vi "phasemap_slope.vi"() -> ()   [LabVIEW 2011]
uses:
  global_vars.vi
  <userlib>/_OpenG.lib/file/file.llb/Build Path - Traditional__ogtk.vi
panel:
  out "select_col 2":dbl[](array[numeric])
  out "check1":dbl[][](array[numeric])
  out "select_col":dbl[](array[numeric])
  in  "pick col":i32(slide)=225 min=0 scale=0.0..999.0
  out "Y_Displacement (px)":i32[](graph)
  out "X_Displacement (px)":i32[](graph)
  out "x_px_dist":i32[](array[numeric])
  out "Min_values":dbl[](array[numeric])
  out "Min_indices":dbl[](array[numeric])
  out "M_test":dbl[][](array[numeric])
  out "u8_ar_phase map 2":u8[][](array[numeric])
  out "nd_ar_unwrapped_px_ar":dbl[][](array[numeric])
  out "df_ar_unwrapped_px_ar":dbl[][](array[numeric])
  out "Ndist_img":u8[][][](array[numeric])
  in  "read files no-dist":bool
  in  "normalize":bool=TRUE
  out "Phase Line (unwrapped)":dbl[](graph)=[0.0, 0.6594827586206897, 1.0991379310344829, 1.3189655172413794, 1.978448275862069, 2.418103448275862, 2.8577586206896552, 3.2974137931034484, 3.7370689655172415, 4.176724137931035, 4.616379310344827, 5.056034482758621, 5.495689655172414, 5.935344827586207, 6.375, 6.814655172413794, 7.254310344827586, 7.69396551724138, 8.133620689655173, 8.573275862068966, 9.01293103448276, 9.452586206896552, 9.892241379310345, 10.331896551724139, 10.551724137931036, 10.991379310344827, 11.431034482758621, 11.870689655172415, 12.310344827586208, 12.75, 13.189655172413794, 13.629310344827587, 14.068965517241379, 14.508620689655173, 14.948275862068966, 15.38793103448276, 15.607758620689657, 16.04741379310345, 16.487068965517242, 16.926724137931036, 17.36637931034483, 17.806034482758623, 18.02586206896552, 18.46551724137931, 18.905172413793103, 19.344827586206897, 19.78448275862069, 20.224137931034484, 20.44396551724138, 21.10344827586207, 21.323275862068968, 21.762931034482758, 22.20258620689655, 22.642241379310345, 22.862068965517242, 23.301724137931036, 23.74137931034483, 24.181034482758623, 24.620689655172416, 24.84051724137931, 25.280172413793103, 25.719827586206897, 26.15948275862069, 26.379310344827587, 26.81896551724138, 27.258620689655174, 27.47844827586207, 27.918103448275865, 28.357758620689655, 28.57758620689655, 29.017241379310345, 29.45689655172414, 29.896551724137932, 30.11637931034483, 30.556034482758623, 30.995689655172416, 31.435344827586206, 31.655172413793103, 32.0948275862069, 32.314655172413794, 32.75431034482759, 33.19396551724138, 33.41379310344828, 33.85344827586207, 34.293103448275865, 34.51293103448276, 34.952586206896555, 35.39224137931035, 35.612068965517246, 36.05172413793104, 36.491379310344826, 36.71120689655172, 37.150862068965516, 37.37068965517241, 37.810344827586206, 38.25, 38.4698275862069, 38.90948275862069, 39.12931034482759, 39.56896551724138, 40.008620689655174, 40.22844827586207, 40.668103448275865, 40.88793103448276, 41.327586206896555, 41.54741379310345, 41.987068965517246, 42.42672413793104, 42.646551724137936, 42.86637931034483, 43.30603448275862, 43.74568965517241, 43.96551724137931, 44.4051724137931, 44.625, 45.064655172413794, 45.28448275862069, 45.724137931034484, 45.94396551724138, 46.383620689655174, 46.60344827586207, 47.043103448275865, 47.26293103448276, 47.702586206896555, 47.92241379310345, 48.362068965517246, 48.58189655172414, 49.021551724137936, 49.24137931034483, 49.46120689655173, 49.900862068965516, 50.12068965517241, 50.560344827586206, 50.7801724137931, 51.2198275862069, 51.439655172413794, 51.87931034482759, 52.099137931034484, 52.53879310344828, 52.758620689655174, 52.97844827586207, 53.418103448275865, 53.63793103448276, 54.077586206896555, 54.29741379310345, 54.51724137931035, 54.95689655172414, 55.17672413793104, 55.396551724137936, 55.83620689655173, 56.056034482758626, 56.49568965517241, 56.71551724137931, 57.1551724137931, 57.375, 57.5948275862069, 57.814655172413794, 58.25431034482759, 58.474137931034484, 58.69396551724138, 59.133620689655174, 59.35344827586207, 59.793103448275865, 60.01293103448276, 60.23275862068966, 60.67241379310345, 60.89224137931035, 61.112068965517246, 61.33189655172414, 61.771551724137936, 61.99137931034483, 62.431034482758626, 62.65086206896552, 62.87068965517241, 63.09051724137931, 63.310344827586206, 63.75, 63.9698275862069, 64.1896551724138, 64.62931034482759, 64.84913793103449, 65.06896551724138, 65.28879310344828, 65.72844827586208, 65.94827586206897, 66.16810344827586, 66.60775862068965, 66.82758620689656, 67.04741379310344, 67.26724137931035, 67.48706896551724, 67.92672413793103, 68.14655172413794, 68.36637931034483, 68.58620689655173, 68.80603448275862, 69.24568965517241, 69.46551724137932, 69.6853448275862, 69.90517241379311, 70.125, 70.5646551724138, 70.7844827586207, 71.00431034482759, 71.22413793103449, 71.66379310344828, 71.88362068965517, 72.10344827586208, 72.32327586206897, 72.54310344827587, 72.76293103448276, 73.20258620689656, 73.42241379310344, 73.64224137931035, 73.86206896551724, 74.08189655172414, 74.30172413793103, 74.74137931034483, 74.96120689655173, 75.18103448275862, 75.40086206896552, 75.62068965517241, 75.84051724137932, 76.0603448275862, 76.5, 76.7198275862069, 76.9396551724138, 77.1594827586207, 77.37931034482759, 77.59913793103449, 77.81896551724138, 78.03879310344828, 78.25862068965517, 78.47844827586208, 78.91810344827587, 79.13793103448276, 79.13793103448276, 79.57758620689656, 79.79741379310344, 80.01724137931035, 80.23706896551724, 80.45689655172414, 80.67672413793103, 80.89655172413794, 81.11637931034483, 81.33620689655173, 81.55603448275862, 81.77586206896552, 82.21551724137932, 82.4353448275862, 82.65517241379311, 82.875, 83.0948275862069, 83.3146551724138, 83.5344827586207, 83.75431034482759, 83.97413793103449, 84.19396551724138, 84.41379310344828, 84.63362068965517, 84.85344827586208, 85.07327586206897, 85.29310344827587, 85.51293103448276, 85.73275862068967, 85.73275862068967, 85.95258620689656, 86.17241379310344, 86.39224137931035, 86.61206896551724, 86.83189655172414, 87.05172413793103, 87.27155172413794, 87.49137931034483, 87.71120689655173, 87.93103448275862, 88.15086206896552, 88.37068965517241, 88.59051724137932, 88.8103448275862, 89.03017241379311, 89.25, 89.4698275862069, 89.6896551724138, 89.9094827586207, 90.12931034482759, 90.34913793103449, 90.56896551724138, 90.78879310344828, 91.00862068965517, 91.22844827586208, 91.44827586206897, 91.44827586206897, 91.88793103448276, 91.88793103448276, 92.32758620689656, 92.54741379310344, 92.54741379310344, 92.76724137931035, 92.98706896551724, 93.20689655172414, 93.42672413793103, 93.64655172413794, 93.86637931034483, 94.08620689655173, 94.30603448275862, 94.52586206896552, 94.52586206896552, 94.96551724137932, 94.96551724137932, 95.1853448275862, 95.40517241379311, 95.625, 95.8448275862069, 96.0646551724138, 96.2844827586207, 96.50431034482759, 96.72413793103449, 96.72413793103449, 96.94396551724138, 97.16379310344828, 97.38362068965517, 97.60344827586208, 97.82327586206897, 98.04310344827587, 98.26293103448276, 98.48275862068967, 98.48275862068967, 98.70258620689656, 98.92241379310346, 99.14224137931035, 99.36206896551724, 99.58189655172414, 99.80172413793103, 100.02155172413794, 100.02155172413794, 100.24137931034483, 100.46120689655173, 100.68103448275862, 100.90086206896552, 101.12068965517241, 101.34051724137932, 101.34051724137932, 101.5603448275862, 101.78017241379311, 102.0, 102.2198275862069, 102.4396551724138, 102.4396551724138, 102.6594827586207, 102.87931034482759, 103.09913793103449, 103.31896551724138, 103.53879310344828, 103.53879310344828, 103.75862068965517, 103.97844827586208, 104.19827586206897, 104.41810344827587, 104.63793103448276, 104.63793103448276, 104.85775862068967, 105.07758620689656, 105.29741379310346, 105.29741379310346, 105.51724137931035, 105.73706896551724, 105.95689655172414, 106.17672413793103, 106.39655172413794, 106.61637931034483, 106.61637931034483, 106.83620689655173, 107.05603448275862, 107.05603448275862, 107.27586206896552, 107.49568965517241, 107.71551724137932, 107.9353448275862, 108.15517241379311, 108.375, 108.375, 108.5948275862069, 108.8146551724138, 109.0344827586207, 109.0344827586207, 109.25431034482759, 109.47413793103449, 109.69396551724138, 109.91379310344828, 109.91379310344828, 110.13362068965517, 110.35344827586208, 110.57327586206897, 110.57327586206897, 110.79310344827587, 111.01293103448276, 111.23275862068967, 111.23275862068967, 111.45258620689656, 111.67241379310346, 111.89224137931035, 112.11206896551725, 112.11206896551725, 112.33189655172414, 112.55172413793103, 112.77155172413794, 112.99137931034483, 112.99137931034483, 113.21120689655173, 113.43103448275862, 113.43103448275862, 113.65086206896552, 113.87068965517241, 114.09051724137932, 114.3103448275862, 114.3103448275862, 114.53017241379311, 114.75, 114.75, 114.9698275862069, 115.1896551724138, 115.4094827586207, 115.4094827586207, 115.62931034482759, 115.84913793103449, 116.06896551724138, 116.28879310344828, 116.28879310344828, 116.50862068965517, 116.72844827586208, 116.72844827586208, 116.94827586206897, 117.16810344827587, 117.38793103448276, 117.38793103448276, 117.60775862068967, 117.82758620689656, 117.82758620689656, 118.26724137931035, 118.26724137931035, 118.48706896551725, 118.70689655172414, 118.70689655172414, 118.92672413793103, 118.92672413793103, 119.14655172413794, 119.36637931034483, 119.58620689655173, 119.80603448275862, 119.80603448275862, 120.02586206896552, 120.24568965517241, 120.46551724137932, 120.46551724137932, 120.6853448275862, 120.90517241379311, 120.90517241379311, 121.125, 121.3448275862069, 121.5646551724138, 121.5646551724138, 121.7844827586207, 122.00431034482759, 122.22413793103449, 122.22413793103449, 122.44396551724138, 122.66379310344828, 122.66379310344828, 122.88362068965517, 123.10344827586208, 123.32327586206897, 123.32327586206897, 123.54310344827587, 123.76293103448276, 123.76293103448276, 123.98275862068967, 124.20258620689656, 124.20258620689656, 124.42241379310346, 124.64224137931035, 124.86206896551725, 124.86206896551725, 125.08189655172414, 125.30172413793105, 125.30172413793105, 125.52155172413794, 125.74137931034483, 125.96120689655173, 125.96120689655173, 126.18103448275862, 126.40086206896552, 126.62068965517241, 126.62068965517241, 126.84051724137932, 127.0603448275862, 127.28017241379311, 127.28017241379311, 127.5, 127.5, 127.7198275862069, 127.9396551724138, 128.1594827586207, 128.1594827586207, 128.3793103448276, 128.59913793103448, 128.8189655172414, 128.8189655172414, 129.03879310344828, 129.25862068965517, 129.25862068965517, 129.47844827586206, 129.69827586206898, 129.91810344827587, 129.91810344827587, 130.13793103448276, 130.35775862068965, 130.57758620689657, 130.57758620689657, 130.79741379310346, 130.79741379310346, 131.01724137931035, 131.23706896551724, 131.45689655172416, 131.45689655172416, 131.67672413793105, 131.89655172413794, 132.11637931034483, 132.11637931034483, 132.33620689655172, 132.55603448275863, 132.55603448275863, 132.77586206896552, 132.9956896551724, 133.2155172413793, 133.2155172413793, 133.43534482758622, 133.6551724137931, 133.6551724137931, 133.875, 134.0948275862069, 134.3146551724138, 134.3146551724138, 134.5344827586207, 134.7543103448276, 134.7543103448276, 134.97413793103448, 135.1939655172414, 135.41379310344828, 135.41379310344828, 135.63362068965517, 135.85344827586206, 136.07327586206898, 136.07327586206898, 136.29310344827587, 136.51293103448276, 136.51293103448276, 136.73275862068965, 136.95258620689657, 137.17241379310346, 137.17241379310346, 137.39224137931035, 137.61206896551724, 137.83189655172416, 138.05172413793105, 138.05172413793105, 138.27155172413794, 138.49137931034483, 138.71120689655172, 138.71120689655172, 138.93103448275863, 139.15086206896552, 139.15086206896552, 139.3706896551724, 139.5905172413793, 139.81034482758622, 139.81034482758622, 140.0301724137931, 140.25, 140.25, 140.4698275862069, 140.6896551724138, 140.9094827586207, 141.1293103448276, 141.1293103448276, 141.34913793103448, 141.5689655172414, 141.78879310344828, 141.78879310344828, 142.00862068965517, 142.22844827586206, 142.44827586206898, 142.44827586206898, 142.66810344827587, 142.88793103448276, 143.10775862068965, 143.10775862068965, 143.32758620689657, 143.54741379310346, 143.76724137931035, 143.76724137931035, 143.98706896551724, 144.20689655172416, 144.42672413793105, 144.64655172413794, 144.64655172413794, 144.86637931034483, 145.08620689655174, 145.08620689655174, 145.30603448275863, 145.52586206896552, 145.7456896551724, 145.9655172413793, 146.18534482758622, 146.18534482758622, 146.4051724137931, 146.625, 146.8448275862069, 147.0646551724138, 147.0646551724138, 147.2844827586207, 147.5043103448276, 147.5043103448276, 147.72413793103448, 147.9439655172414, 148.16379310344828, 148.38362068965517, 148.60344827586206, 148.60344827586206, 148.82327586206898, 149.04310344827587, 149.26293103448276, 149.48275862068965, 149.48275862068965, 149.70258620689657, 149.92241379310346, 150.14224137931035, 150.36206896551724, 150.36206896551724, 150.58189655172416, 150.80172413793105, 151.02155172413794, 151.24137931034483, 151.24137931034483, 151.46120689655174, 151.68103448275863, 151.90086206896552, 152.1206896551724, 152.3405172413793, 152.56034482758622, 152.56034482758622, 152.7801724137931, 153.0, 153.2198275862069, 153.4396551724138, 153.6594827586207, 153.6594827586207, 153.8793103448276, 154.09913793103448, 154.3189655172414, 154.53879310344828, 154.75862068965517, 154.75862068965517, 154.97844827586206, 155.19827586206898, 155.41810344827587, 155.63793103448276, 155.85775862068965, 156.07758620689657, 156.07758620689657, 156.29741379310346, 156.51724137931035, 156.73706896551724, 156.95689655172416, 157.17672413793105, 157.39655172413794, 157.61637931034483, 157.83620689655174, 158.05603448275863, 158.27586206896552, 158.4956896551724, 158.4956896551724, 158.7155172413793, 158.93534482758622, 159.1551724137931, 159.375, 159.5948275862069, 159.5948275862069, 159.8146551724138, 160.0344827586207, 160.2543103448276, 160.47413793103448, 160.6939655172414, 160.91379310344828, 161.13362068965517, 161.35344827586206, 161.57327586206898, 161.79310344827587, 162.01293103448276, 162.01293103448276, 162.23275862068965, 162.45258620689657, 162.67241379310346, 162.89224137931035, 163.11206896551724, 163.33189655172416, 163.55172413793105, 163.77155172413794, 163.99137931034483, 164.21120689655174, 164.43103448275863, 164.65086206896552, 164.8706896551724, 165.0905172413793, 165.0905172413793, 165.31034482758622, 165.75, 165.9698275862069, 166.1896551724138, 166.1896551724138, 166.4094827586207, 166.6293103448276, 166.84913793103448, 167.0689655172414, 167.28879310344828, 167.50862068965517, 167.72844827586206, 167.94827586206898, 168.16810344827587, 168.38793103448276, 168.60775862068965, 168.82758620689657, 169.04741379310346, 169.26724137931035, 169.48706896551724, 169.70689655172416, 169.92672413793105, 170.14655172413794, 170.58620689655174, 170.58620689655174, 170.80603448275863, 171.02586206896552, 171.2456896551724, 171.68534482758622, 171.9051724137931, 172.125, 172.3448275862069, 172.5646551724138, 172.7844827586207, 173.0043103448276, 173.22413793103448, 173.4439655172414, 173.66379310344828, 173.88362068965517, 174.10344827586206, 174.32327586206898, 174.54310344827587, 174.76293103448276, 174.98275862068965, 175.20258620689657, 175.64224137931035, 175.64224137931035, 176.08189655172416, 176.30172413793105, 176.52155172413794, 176.74137931034483, 176.96120689655174, 177.18103448275863, 177.40086206896552, 177.6206896551724, 177.84051724137933, 178.2801724137931, 178.5, 178.7198275862069, 178.9396551724138, 179.1594827586207, 179.3793103448276, 179.59913793103448, 179.8189655172414, 180.03879310344828, 180.25862068965517, 180.69827586206898, 180.91810344827587, 181.13793103448276, 181.35775862068965, 181.57758620689657, 181.79741379310346, 182.23706896551724, 182.45689655172416, 182.67672413793105, 182.89655172413794, 183.11637931034483, 183.55603448275863, 183.77586206896552, 183.9956896551724, 184.21551724137933, 184.43534482758622, 184.875, 185.0948275862069, 185.3146551724138, 185.5344827586207, 185.7543103448276, 185.97413793103448, 186.41379310344828, 186.63362068965517, 186.85344827586206, 187.07327586206898, 187.29310344827587, 187.73275862068965, 187.95258620689657, 188.17241379310346, 188.39224137931035, 188.83189655172416, 189.05172413793105, 189.27155172413794, 189.49137931034483, 189.71120689655174, 190.15086206896552, 190.3706896551724, 190.59051724137933, 191.0301724137931, 191.25, 191.4698275862069, 191.6896551724138, 192.1293103448276, 192.34913793103448, 192.5689655172414, 192.78879310344828, 193.22844827586206, 193.44827586206898, 193.66810344827587, 194.10775862068965, 194.32758620689657, 194.76724137931035, 194.98706896551724, 195.20689655172416, 195.42672413793105, 195.86637931034483, 196.08620689655174, 196.30603448275863, 196.7456896551724, 196.96551724137933, 197.18534482758622, 197.625, 197.625, 197.84482758620692, 198.2844827586207, 198.5043103448276, 198.9439655172414, 199.16379310344828, 199.38362068965517, 199.82327586206898, 200.04310344827587, 200.26293103448276, 200.70258620689657, 200.92241379310346, 201.14224137931035, 201.58189655172416, 201.80172413793105, 202.24137931034483, 202.46120689655174, 202.90086206896552, 203.1206896551724, 203.34051724137933, 203.7801724137931, 204.0, 204.4396551724138, 204.6594827586207, 205.09913793103448, 205.3189655172414, 205.75862068965517, 205.97844827586206, 206.19827586206898, 206.63793103448276, 206.85775862068965, 207.29741379310346, 207.73706896551724, 207.95689655172416, 208.17672413793105, 208.61637931034483, 208.83620689655174, 209.27586206896552, 209.4956896551724, 209.93534482758622, 210.1551724137931, 210.59482758620692, 210.8146551724138, 211.2543103448276, 211.47413793103448, 211.91379310344828, 212.13362068965517, 212.57327586206898, 212.79310344827587, 213.23275862068965, 213.67241379310346, 213.89224137931035, 214.33189655172416, 214.55172413793105, 214.99137931034483, 215.43103448275863, 215.65086206896552, 216.09051724137933, 216.31034482758622, 216.75, 216.96982758620692, 217.4094827586207, 217.8491379310345, 218.0689655172414, 218.50862068965517, 218.72844827586206, 219.16810344827587, 219.60775862068965, 219.82758620689657, 220.26724137931035, 220.48706896551724, 220.92672413793105, 221.36637931034483, 221.80603448275863, 222.02586206896552, 222.46551724137933, 222.68534482758622, 223.125, 223.5646551724138, 223.7844827586207, 224.2241379310345, 224.66379310344828, 224.88362068965517, 225.32327586206898, 225.76293103448276, 226.20258620689657, 226.42241379310346, 226.86206896551724, 227.30172413793105, 227.52155172413794, 227.96120689655174, 228.40086206896552, 228.84051724137933, 229.06034482758622, 229.5, 229.9396551724138, 230.3793103448276, 230.5991379310345, 231.03879310344828, 231.47844827586206, 231.91810344827587, 232.35775862068965, 232.57758620689657, 233.01724137931035, 233.45689655172416, 233.89655172413794, 234.33620689655174, 234.55603448275863, 234.9956896551724, 235.43534482758622, 235.875, 236.09482758620692, 236.5344827586207, 236.9741379310345, 237.41379310344828, 237.85344827586206, 238.29310344827587, 238.73275862068965, 239.17241379310346, 239.39224137931035, 239.83189655172416, 240.27155172413794, 240.71120689655174, 241.15086206896552, 241.59051724137933, 242.0301724137931, 242.46982758620692, 242.6896551724138, 243.1293103448276, 243.5689655172414, 244.00862068965517, 244.44827586206898, 244.88793103448276, 245.32758620689657, 245.76724137931035, 246.20689655172416, 246.64655172413794, 247.08620689655174, 247.52586206896552, 247.96551724137933, 248.4051724137931, 248.84482758620692, 249.2844827586207, 249.7241379310345, 250.16379310344828, 250.6034482758621, 251.04310344827587, 251.48275862068965, 251.92241379310346, 252.36206896551724, 252.80172413793105, 253.24137931034483, 253.68103448275863, 254.1206896551724, 254.56034482758622, 255.0]
  out "u8_ar_phase map":u8[][](array[numeric])
  in  "pick row":i32(slide)=225 min=0 scale=0.0..499.0
  in  "calculate \nphase map":bool
  out "img_phase map":T1(plugin-control)
  out "current image":T1(plugin-control)
  out "Dist_img":u8[][][](array[numeric])
  in  "current image":string="fringe"
  in  "pick input image":i32
  in  "phase map file name":string="orig.png"
  in  "EXP Folder Path":path=path "X:/Cloud Drives/Dropbox/Europhotonics/FringeMan/Image Storage/01_09/playing around" caption="Enter or select file path"
  in  "save phasemap":bool
  in  "read files":bool
  in  "Stop Button":bool
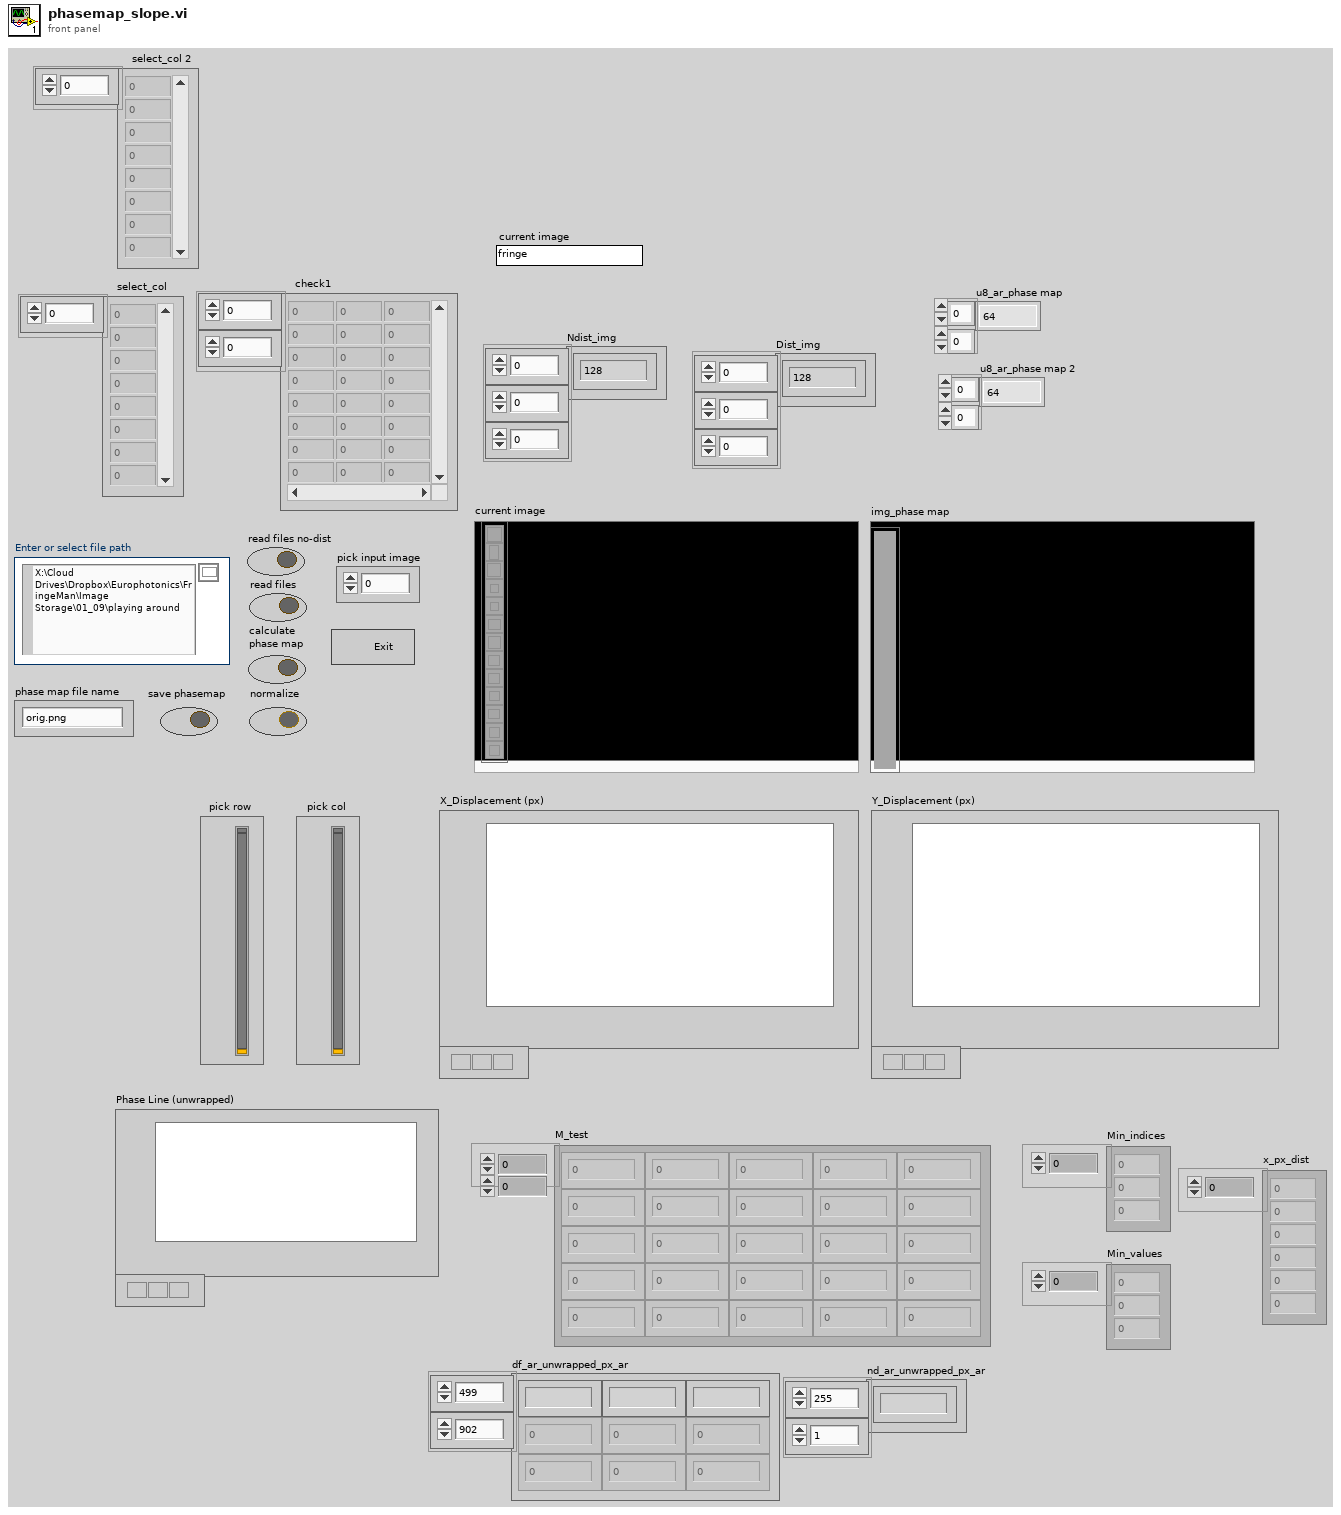
[diagram p1: front panel]
types:
  T1 = typedef "IMAQ Image.ctl" = refnum<image>
  T2 = typedef "Image Type" = u32
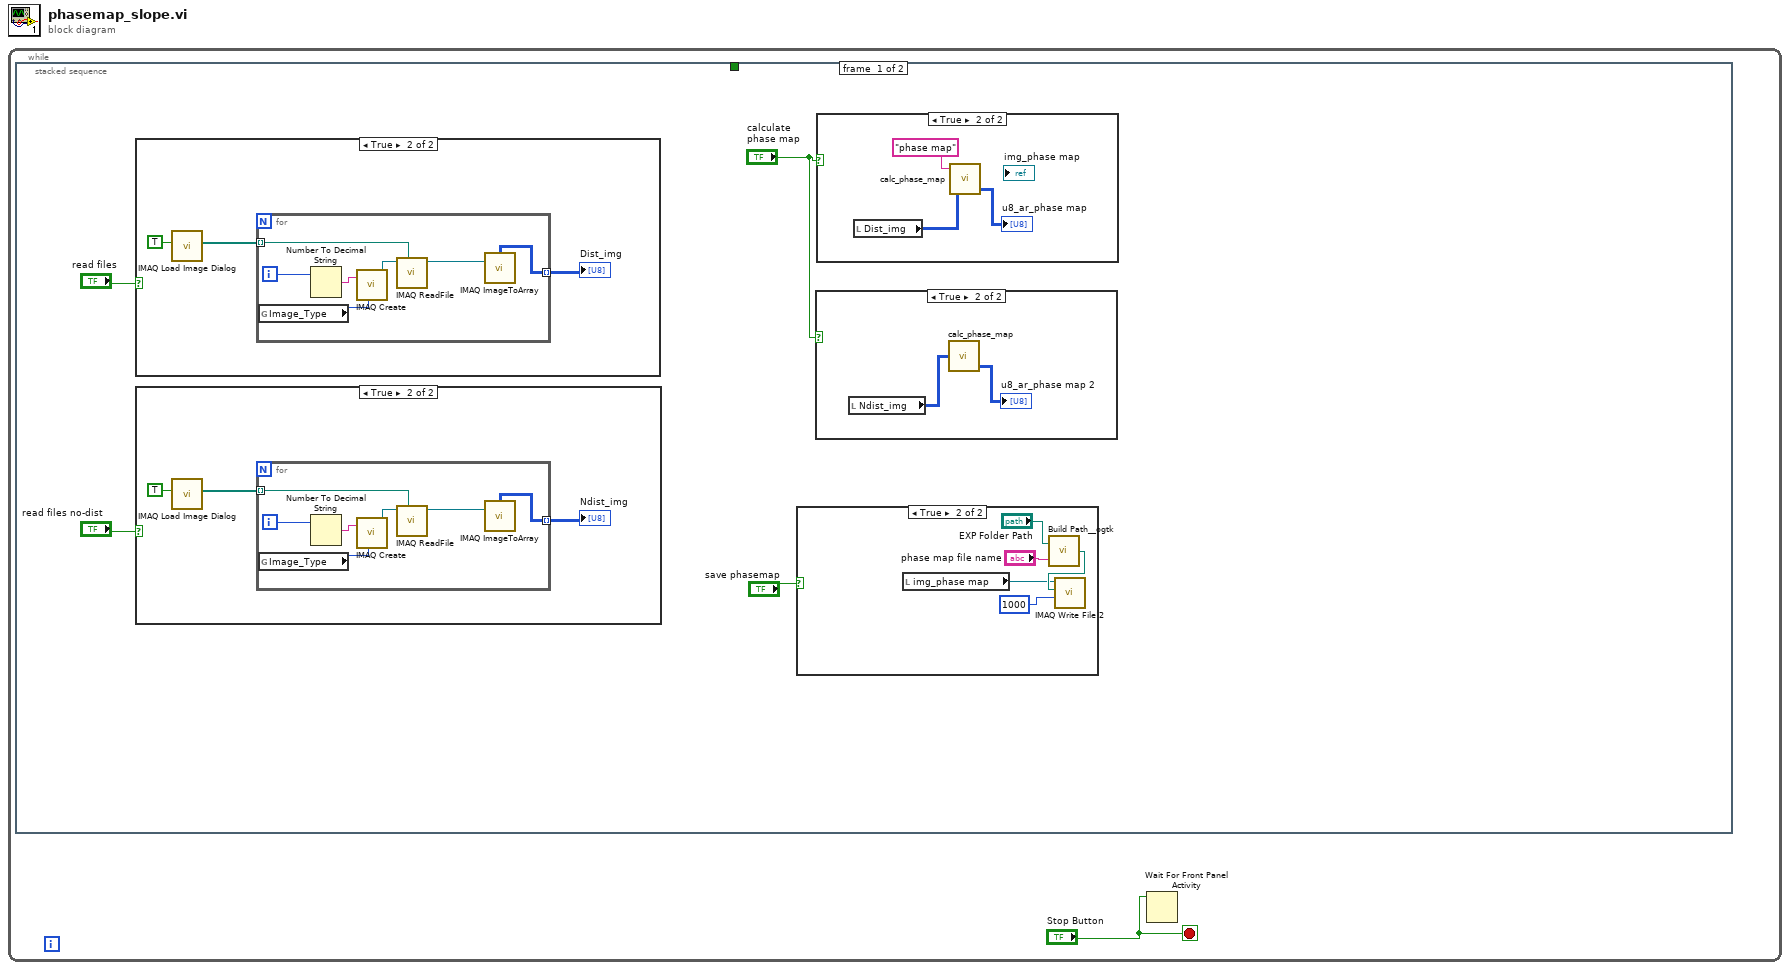
[diagram p0: block diagram]
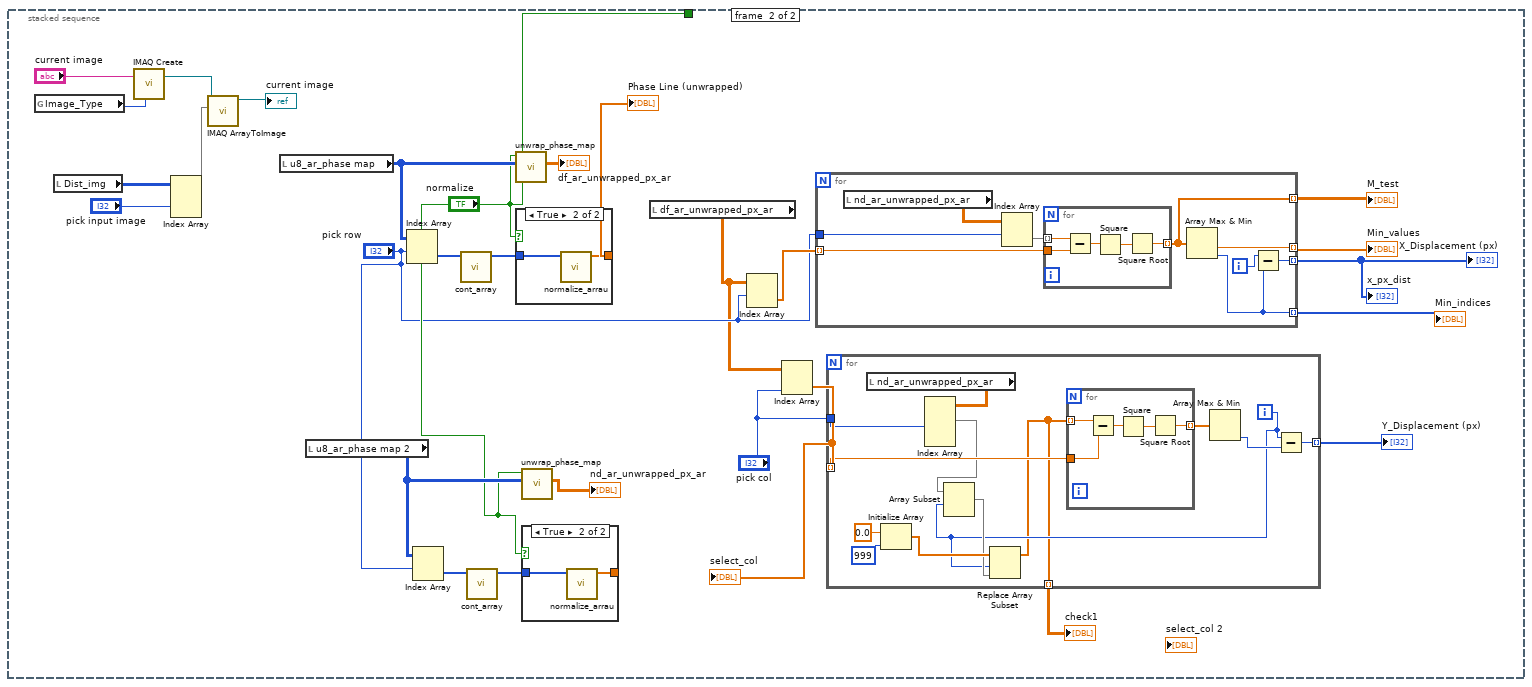
[diagram p7: hidden frame]
diagram:
  n1 = while {
    stop <- "Stop Button" stop-if-true
    n2 = stacked-sequence {
      tunnel: [_ "normalize"] -> _
      frame #0 {
        n3 = case shown="True" "read files" {
          frame False {
          }
          frame True {
            n4 = call "IMAQ Load Image Dialog"("Multiple Files? (No)"=TRUE) -> ("Paths"=w28:path[])  [unwired: 8 in, 2 out]
            n5 = for {
              tunnel: w28 -> [w35] mode=indexing
              tunnel: [w30] -> w26 mode=indexing
              i -> [w34]
              n6 = global read "global_vars.vi" "Image_Type"() -> (w29:T2)
              n7 = Number To Decimal String(number=w34) -> (decimal integer string=w33:string)  [unwired: 1 in]
              n8 = call "IMAQ Create"("Image Name"=w33, "Image Type"=w29) -> ("New Image"=w32:T1)  [unwired: 2 in, 2 out]
              n9 = call "IMAQ ReadFile"("File Path"=w35, "Image"=w32) -> ("Image Out"=w31:T1)  [unwired: 5 in, 4 out]
              n10 = call "IMAQ ImageToArray"("Image"=w31) -> ("Image Pixels (U8)"=w30:u8[][])  [unwired: 3 in, 4 out]
            }
            "Dist_img" <- w26
          }
        }
        n11 = case shown="True" "read files no-dist" {
          frame False {
          }
          frame True {
            n12 = call "IMAQ Load Image Dialog"("Multiple Files? (No)"=TRUE) -> ("Paths"=w10:path[])  [unwired: 8 in, 2 out]
            n13 = for {
              tunnel: w10 -> [w17] mode=indexing
              tunnel: [w13] -> w8 mode=indexing
              i -> [w11]
              n14 = global read "global_vars.vi" "Image_Type"() -> (w12:T2)
              n15 = Number To Decimal String(number=w11) -> (decimal integer string=w16:string)  [unwired: 1 in]
              n16 = call "IMAQ Create"("Image Name"=w16, "Image Type"=w12) -> ("New Image"=w15:T1)  [unwired: 2 in, 2 out]
              n17 = call "IMAQ ReadFile"("File Path"=w17, "Image"=w15) -> ("Image Out"=w14:T1)  [unwired: 5 in, 4 out]
              n18 = call "IMAQ ImageToArray"("Image"=w14) -> ("Image Pixels (U8)"=w13:u8[][])  [unwired: 3 in, 4 out]
            }
            "Ndist_img" <- w8
          }
        }
        n19 = case shown="True" "save phasemap" {
          frame False {
          }
          frame True {
            n20 = local read "img_phase map"() -> (w21:T1)
            n21 = call-poly <userlib>:"Build Path__ogtk.vi"("name or relative path"="phase map file name", "base path"="EXP Folder Path") -> ("appended path"=w23:path)
            n22 = call-poly "IMAQ Write File 2"("Image Quality"=u32 1000, "File Path"=w23, "Image"=w21) -> ()  [unwired: 7 in, 2 out]
          }
        }
        n23 = case shown="True" "calculate \nphase map" {
          frame False {
          }
          frame True {
            n24 = local read "Ndist_img"() -> (w6:u8[][][])
            n25 = call "calc_phase_map.vi"("u8_ar_image_pixel_array"=w6) -> ("raw phase map array"=→"u8_ar_phase map 2":u8[][])  [unwired: 3 in, 1 out]
          }
        }
        n26 = case shown="True" "calculate \nphase map" {
          frame False {
          }
          frame True {
            n27 = local read "Dist_img"() -> (w19:u8[][][])
            n28 = call "calc_phase_map.vi"("u8_ar_image_pixel_array"=w19, "image name"="phase map" ("String")) -> ("raw phase map array"=→"u8_ar_phase map":u8[][])  [unwired: 2 in, 1 out]
          }
        }
      }
      frame #1 {
        n29 = global read "global_vars.vi" "Image_Type"() -> (w60:T2)
        n30 = local read "Dist_img"() -> (w63:u8[][][])
        n31 = call "IMAQ Create"("Image Name"="current image", "Image Type"=w60) -> ("New Image"=w62:T1)  [unwired: 2 in, 2 out]
        n32 = Index Array(array=w63, index (dim 0)="pick input image") -> (element=w57:u8[][])  [unwired: 2 in]
        n33 = call "IMAQ ArrayToImage"("Image Pixels (U8)"=w57, "Image"=w62) -> ("Image Out"=→"current image":T1)  [unwired: 8 in, 1 out]
        n34 = local read "u8_ar_phase map"() -> (w55:u8[][])
        n35 = local read "u8_ar_phase map 2"() -> (w51:u8[][])
        n36 = Index Array(array=w55, index (row)="pick row") -> (element=w56:u8[])  [unwired: 1 in]
        n37 = Index Array(array=w51, index (row)="pick row") -> (element=w50:u8[])  [unwired: 1 in]
        n38 = call "cont_array.vi"("u8_ar_phase map"=w56) -> ("Array"=w54:i16[])  [unwired: 10 in]
        n39 = call "cont_array.vi"("u8_ar_phase map"=w50) -> ("Array"=w52:i16[])  [unwired: 10 in]
        n40 = call "unwrap_phase_map.vi"("u8_ar_phase map"=w55, "normalize (y)"="normalize") -> ("df_ar_unwrapped_px_ar"=→"df_ar_unwrapped_px_ar":dbl[][])  [unwired: 8 in, 1 out]
        n41 = case shown="True" "normalize" {
          tunnel: w54 -> [w99 w101]
          tunnel: [w99 w100] -> w53
          frame False {
          }
          frame True {
            n42 = call "normalize_arrau.vi"("Array in"=w101) -> ("Array out"=w100:dbl[])  [unwired: 10 in]
          }
        }
        "Phase Line (unwrapped)" <- w53
        n43 = call "unwrap_phase_map.vi"("u8_ar_phase map"=w51, "normalize (y)"="normalize") -> ("df_ar_unwrapped_px_ar"=→"nd_ar_unwrapped_px_ar":dbl[][])  [unwired: 8 in, 1 out]
        n44 = case shown="True" "normalize" {
          tunnel: w52 -> [w96 w98]
          tunnel: [w96 w97] -> _
          frame False {
          }
          frame True {
            n45 = call "normalize_arrau.vi"("Array in"=w98) -> ("Array out"=w97:dbl[])  [unwired: 10 in]
          }
        }
        n46 = local read "df_ar_unwrapped_px_ar"() -> (w38:dbl[][])
        n47 = Index Array(array=w38, index (row)="pick row") -> (element=w47:dbl[])  [unwired: 1 in]
        n48 = Index Array(array=w38, index (col)="pick col") -> (element=w37:dbl[])  [unwired: 1 in]
        "select_col" <- w37
        n49 = for {
          tunnel: w47 -> [w87] mode=indexing
          tunnel: "pick row" -> [w89]
          tunnel: [w86] -> w44 mode=indexing
          tunnel: [w82] -> w46 mode=indexing
          tunnel: [w85] -> w45 mode=indexing
          tunnel: [w84] -> w43 mode=indexing
          i -> [w83]
          n50 = local read "nd_ar_unwrapped_px_ar"() -> (w90:dbl[][])
          n51 = Index Array(array=w90, index (row)=w89) -> (element=w88:dbl[])  [unwired: 1 in]
          n52 = for {
            tunnel: w88 -> [w95] mode=indexing
            tunnel: w87 -> [w94]
            tunnel: [w91] -> w86 mode=indexing
            n53 = Subtract(x=w95, y=w94) -> (x-y=w93:dbl)
            n54 = Square(x=w93) -> (x^2=w92:dbl)
            n55 = Square Root(x=w92) -> (sqrt(x)=w91:dbl)
          }
          n56 = Array Max & Min(array=w86) -> (min value=w85:dbl, min index (indices)=w82:i32)  [unwired: 2 out]
          n57 = Subtract(x=w83, y=w82) -> (x-y=w84:i32)
        }
        "M_test" <- w44
        "Min_indices" <- w46
        "Min_values" <- w45
        "x_px_dist" <- w43
        "X_Displacement (px)" <- w43
        n58 = for {
          tunnel: w37 -> [w75] mode=indexing
          tunnel: [w73] -> w40 mode=indexing
          tunnel: "pick col" -> [w72]
          tunnel: [w64] -> w36 mode=indexing
          i -> [w65]
          n59 = local read "nd_ar_unwrapped_px_ar"() -> (w76:dbl[][])
          n60 = Initialize Array(0.0 ("element"), 999 ("dimension size")) -> (w67:dbl[])
          n61 = Index Array(array=w76, index (col) #1=w72) -> (element #1=w70:dbl[])  [unwired: 3 in, 1 out]
          n62 = Array Subset(array=w70, index=w65) -> (w66:dbl[])  [unwired: 1 in]
          n63 = Replace Array Subset(array=w67, new element=w66, index=w65) -> (w64:dbl[])
          n64 = for {
            tunnel: w75 -> [w81]
            tunnel: [w78] -> w74 mode=indexing
            tunnel: w64 -> [w77] mode=indexing
            n65 = Subtract(x=w77, y=w81) -> (x-y=w80:dbl)
            n66 = Square(x=w80) -> (x^2=w79:dbl)
            n67 = Square Root(x=w79) -> (sqrt(x)=w78:dbl)
          }
          n68 = Array Max & Min(array=w74) -> (min index (indices)=w71:i32)  [unwired: 3 out]
          n69 = Subtract(x=w65, y=w71) -> (x-y=w73:i32)
        }
        "Y_Displacement (px)" <- w40
        "check1" <- w36
      }
    }
    n70 = Wait For Front Panel Activity(3:"Stop Button") -> ()  [unwired: 2 in, 1 out]
  }
